vi "UHR-Fleezers Control (host) - 12.7.vi"() -> ()   [LabVIEW 2012] (continued)
        n1557 = Multiply(x=w2182, y="Number of F/B Scans (AOD)") -> (x*y=w2179:dbl)
        n1558 = Divide(x=w2179, y=60.0) -> (x/y=→"Time to Finish All (min)":dbl)
        n1559 = Add(x="Trap 2 Bead Size (nm)", y="Trap 1 Bead Size (nm)") -> (x+y=w2223:dbl)
        n1560 = Divide(x=w2223, y=2.0) -> (x/y=w2217:dbl)
        n1561 = local read "Initial delta (MHz)"() -> (w2220:dbl)
        n1562 = Subtract(x=w2234, y=w2233) -> (x-y=w2231:dbl)
        n1563 = Subtract(x=w2235, y=w2236) -> (x-y=w2232:dbl)
        n1564 = Square(x=w2231) -> (x^2=w2230:dbl)
        n1565 = Square(x=w2232) -> (x^2=w2229:dbl)
        n1566 = Add(x=w2229, y=w2230) -> (x+y=w2228:dbl)
        n1567 = Square Root(x=w2228) -> (sqrt(x)=w2227:dbl)
        "Final delta (MHz)" <- w2227
        n1568 = Multiply(x=w2219, y=w2227) -> (x*y=w2226:dbl)
        n1569 = Multiply(x=w2220, y=w2219) -> (x*y=w2218:dbl)
        n1570 = Subtract(x=w2218, y=w2217) -> (x-y=→"Initial sep (nm)":dbl)
        n1571 = Subtract(x=w2226, y=w2217) -> (x-y=→"Final sep (nm)":dbl)
      }
      event "Freq or Amp switch first", "Swap F1 and F2", "Freq switch delay", "Amp switch delay": Value Change {
        n1572 = event-data() -> ()  [unwired: 7 out]
        n1573 = local read "Amp switch delay"() -> (w2252:u16)
        n1574 = local read "Swap F1 and F2"() -> (w2253:bool)
        n1575 = xnode "Read/Write Control"("FPGA VI Reference In"=w2256, "error in"=w2255, "Swap F1 and F2"=w2253, "Amp switch delay"=w2252) -> ("error out"=w2254:errorcluster)  [unwired: 1 out]
      }
      event "Scan steps (MCL)", "Number of scans (MCL)", "Scan Range (V)\n(of steps)", "2D or 1D Scan", "N APD Samp/step", "Fast Scan Dir", "Continuous MCL Scanning", "Scan lines (y)": Value Change {
        w2258 = 32767.0 ("y")
        n1576 = event-data() -> ()  [unwired: 7 out]
        n1577 = Select(t="Scan lines (y)", s="2D or 1D Scan", f="Number of scans (MCL)") -> (s? t:f=w2263:u64)
        n1578 = Decrement(x="Scan steps (MCL)") -> (x-1=w2279:u64)
        n1579 = Divide(x="Scan Range (V)\n(of steps)", y=w2279) -> (x/y=w2278:dbl)
        "Desired Scan Incr (V)" <- w2278
        n1580 = local read "APD Integration Time (s)"() -> (w2271:dbl)
        n1581 = Multiply(x=w2278, y=w2258) -> (x*y=w2287:dbl)
        n1582 = Divide(x=w2287, y=10.0) -> (x/y=w2277:dbl)
        "Desired incr (int)" <- w2277
        n1583 = local read "Update Count (MCL)"() -> (w2283:u32)
        n1584 = Round Toward -Infinity(1:w2277) -> (0:w2286:dbl)
        n1585 = To Word Integer(number=w2286) -> (16bit integer=w2261:i16)
        "Actual Incr. int (MCL)" <- w2261
        n1586 = Multiply(x=w2271, y=40000000.0) -> (x*y=w2284:dbl)
        n1587 = Divide(x=w2284, y=w2283) -> (x/y=w2282:dbl)
        n1588 = Multiply(x=i16 10, y=w2261) -> (x*y=w2259:i16)
        n1589 = Multiply(x="N APD Samp/step", y=w2282) -> (x*y=w2281:dbl)
        "Cycles/step (MCL)" <- w2281
        n1590 = Divide(x=w2259, y=w2258) -> (x/y=→"Actual MCL Inc (V)":dbl)
        n1591 = Multiply(x="N APD Samp/step", y="Scan steps (MCL)") -> (x*y=w2273:dbl)
        n1592 = local read "APD Samples/FIFO Acq."() -> (w2270:dbl)
        n1593 = Multiply(x=w2273, y=u64 2) -> (x*y=w2272:dbl)
        "Data points/scan (f+b)" <- w2272
        n1594 = Multiply(x=w2272, y=w2263) -> (x*y=w2290:dbl)
        "Data points/scans (MCL)" <- w2290
        n1595 = Multiply(x=w2271, y=w2272) -> (x*y=w2264:dbl)
        "Time/f+b scan (s) (MCL)" <- w2264
        n1596 = Divide(x=w2290, y=w2270) -> (x/y=→"N sets should be saved (MCL)":dbl)
        n1597 = Multiply(x=w2264, y=w2263) -> (x*y=→"Total Time (s)":dbl)
        n1598 = Not(x="Fast Scan Dir") -> (.not. x?=w2268:bool)
        n1599 = xnode "Read/Write Control"("FPGA VI Reference In"=w2294, "error in"=w2293, "Scan steps (MCL)"="Scan steps (MCL)", "Number of scans (MCL)"=w2263, "Cycles per step (MCL)"=w2281, "Scan freq.  increment (MCL)"=w2261, "1D or 2D Scan?"="2D or 1D Scan", "MCL Scan Axis"=w2268, "Cont. Scan (MCL)"="Continuous MCL Scanning") -> ("error out"=w2292:errorcluster)  [unwired: 1 out]
      }
      event "Read Cal": Value Change {
        w2296 = 1000.0 ("y")
        n1600 = event-data() -> ()  [unwired: 7 out]
        n1601 = local read "Save file name"() -> (w2321:path)
        n1602 = local write "Read Cal"(FALSE ("Read Cal")) -> ()
        n1603 = Strip Path(path=w2321) -> (stripped path=w2320:path)  [unwired: 1 out]
        n1604 = Path To String(path=w2320) -> (string=w2319:string)
        n1605 = Concatenate Strings(w2319, "\\current.cal" ("string")) -> (w2317:string)
        n1606 = String To Path(string=w2317) -> (path=w2316:path)
        n1607 = Open/Create/Replace File(file path (use dialog)=w2316, operation (0:open)=T29."open", access (0:read/write)=enum16{"read/write", "read-only", "write-only"}."read-only") -> (refnum out=w2324:refnum<file>, error out=w2310:errorcluster)  [unwired: 1 in, 3 out]
        n1608 = Deny Access(4:w2310, 7:w2324) -> (0:w2309:errorcluster, 3:w2315:refnum<file>)  [unwired: 1 out]
        n1609 = Read from Binary File(5:0.0, 8:w2309, 9:T28."big-endian, network order" ("byte order (0:big-endian, network order)"), 10:-1 ("count (1)"), 11:w2315) -> (0:w2308:errorcluster, 2:w2306:dbl[], 3:w2311:refnum<file>)  [unwired: 2 out]
        n1610 = Array To Cluster(array=w2306) -> (cluster=w2305:T31)
        n1611 = Unbundle(w2305) -> ("[0]"=w2304:dbl, "[1]"=w2303:dbl, "[2]"=w2302:dbl, "[3]"=w2301:dbl, "[4]"=w2300:dbl, "[5]"=w2299:dbl)
        n1612 = Close File(refnum=w2311, error in=w2308) -> (error out=→"Read cal error":errorcluster)  [unwired: 1 out]
        n1613 = Multiply(x=w2299, y=w2296) -> (x*y=w2297:dbl)
        n1614 = local write "T2 kappa_x (pN/nm)"(w2301) -> ()
        n1615 = local write "T1 kappa_x (pN/nm)"(w2302) -> ()
        n1616 = local write "T1 alpha_x (nm/V)"(w2304) -> ()
        n1617 = local write "T2 alpha_x (nm/V)"(w2303) -> ()
        n1618 = Multiply(x=w2300, y=w2296) -> (x*y=w2298:dbl)
        n1619 = local write "T1 offset_x (mV)"(w2298) -> ()
        n1620 = local write "T2 offset_x (mV)"(w2297) -> ()
      }
      event "Abort MCL Scan": Value Change {
        n1621 = event-data() -> ()  [unwired: 7 out]
        n1622 = local write "MCL Scanning"(FALSE ("MCL Scanning")) -> ()
        n1623 = xnode "Read/Write Control"("FPGA VI Reference In"=w2329, "error in"=w2328, "Abort scan (MCL)"="Abort MCL Scan") -> ("error out"=w2327:errorcluster)  [unwired: 1 out]
      }
      event "Update Count (MCL)": Value Change {
        n1624 = event-data() -> ()  [unwired: 7 out]
        n1625 = xnode "Read/Write Control"("FPGA VI Reference In"=w2333, "error in"=w2332, "MCL count"="Update Count (MCL)") -> ("error out"=w2331:errorcluster)  [unwired: 1 out]
      }
      event "+ phase (MCL)", "- phase (MCL)": Value Change {
        n1626 = event-data() -> ()  [unwired: 7 out]
        n1627 = Or(x="- phase (MCL)", y="+ phase (MCL)") -> (x .or. y?=w2336:bool)
        n1628 = Negate(x="Phase adjust (MCL)") -> (-x=w2342:i16)
        n1629 = Select(t=w2342, s="+ phase (MCL)", f="Phase adjust (MCL)") -> (s? t:f=w2340:i16)
        n1630 = xnode "Read/Write Control"("FPGA VI Reference In"=w2344, "error in"=w2343, "Phase count adjustment (MCL)"=w2340) -> ("FPGA VI Reference Out"=w2337:T20, "error out"=w2338:errorcluster)
        n1631 = xnode "Read/Write Control"("FPGA VI Reference In"=w2337, "error in"=w2338, "+ phase (MCL)"=w2336) -> ("error out"=w2335:errorcluster)  [unwired: 1 out]
      }
      event "Abort AOD Scan": Value Change {
        n1632 = event-data() -> ()  [unwired: 7 out]
        n1633 = xnode "Read/Write Control"("FPGA VI Reference In"=w2348, "error in"=w2347, "Abort scan"="Abort AOD Scan") -> ("error out"=w2346:errorcluster)  [unwired: 1 out]
      }
      event "Continuous AOD Scanning": Value Change {
        n1634 = event-data() -> ()  [unwired: 7 out]
        n1635 = xnode "Read/Write Control"("FPGA VI Reference In"=w2352, "error in"=w2351, "Cont. Scan"="Continuous AOD Scanning") -> ("error out"=w2350:errorcluster)  [unwired: 1 out]
      }
      event "Index": Value Change {
        n1636 = event-data() -> ()  [unwired: 7 out]
        n1637 = call "Create new save file.vi"("Insert"="", "Ext"=".dat" ("string"), "Index In"="Index") -> ("Path Out"=→"Save file name":path, "Index Out"=w2353:dbl)
        "Save index" <- w2353
        n1638 = local write "Index"(w2353) -> ()
      }
      event "AO1", "AO2": Value Change {
        w2368 = 10.0 ("y")
        w2367 = 32767.0 ("y")
        n1639 = event-data() -> ()  [unwired: 7 out]
        n1640 = local read "AO2"() -> (w2366:dbl)
        n1641 = local read "AO1"() -> (w2363:dbl)
        n1642 = Multiply(x=w2363, y=w2367) -> (x*y=w2362:dbl)
        n1643 = Multiply(x=w2366, y=w2367) -> (x*y=w2365:dbl)
        n1644 = Divide(x=w2362, y=w2368) -> (x/y=w2361:dbl)
        n1645 = Divide(x=w2365, y=w2368) -> (x/y=w2364:dbl)
        n1646 = To Word Integer(number=w2361) -> (16bit integer=w2369:i16)
        n1647 = To Word Integer(number=w2364) -> (16bit integer=w2370:i16)
        n1648 = xnode "Read/Write Control"("FPGA VI Reference In"=w2360, "error in"=w2359, "AO1"=w2369, "AO2"=w2370) -> ("error out"=w2358:errorcluster)  [unwired: 1 out]
      }
      event "Inject Pump 1": Value Change {
        n1649 = event-data() -> ()  [unwired: 7 out]
        n1650 = local read "Use Harvard pumps\nfor beads (else Chemyx)"() -> (w2372:bool)
        n1651 = case shown="True" w2372 {
          tunnel: "Inject Pump 1" -> [w2376 w2414]
          tunnel: w2371 -> [_ w2415]
          frame False {
            n1652 = local read "Pump write delay (ms)"() -> (w2375:dbl)
            n1653 = local read "Chemyx Syringe Pump Serial Port"() -> (w2374:refnum<visa-resource-name>)
            n1654 = case shown="True" w2376 {
              tunnel: w2375 -> [w2382 w2396]
              tunnel: w2374 -> [w2379 w2395]
              frame False {
                n1655 = flat-sequence {
                  tunnel: w2379 -> [w2383]
                  tunnel: [w2383] -> w2380
                  tunnel: w2382 -> [_]
                  tunnel: [w2386] -> w2381
                  tunnel: w2380 -> [w2386]
                  tunnel: w2381 -> [w2387]
                  tunnel: [w2387] -> w2377
                  tunnel: [w2389] -> w2378
                  tunnel: w2377 -> [w2389]
                  tunnel: w2378 -> [w2391]
                  frame #0 {
                    n1656 = call "Write to pump.vi"("string"="enter pump1", "VISA resource name"=w2383) -> ()  [unwired: 1 out]
                  }
                  frame #1 {
                    n1657 = Wait (ms)(milliseconds to wait="Pump pause delay (ms)") -> ()  [unwired: 1 out]
                  }
                  frame #2 {
                    n1658 = call "Write to pump.vi"("string"="stop", "VISA resource name"=w2387) -> ()  [unwired: 1 out]
                  }
                  frame #3 {
                    n1659 = Wait (ms)(milliseconds to wait=u32 500) -> ()  [unwired: 1 out]
                  }
                  frame #4 {
                    n1660 = call "Write to pump.vi"("string"="stop", "VISA resource name"=w2391) -> ()  [unwired: 1 out]
                  }
                }
              }
              frame True {
                n1661 = flat-sequence {
                  tunnel: w2395 -> [w2405]
                  tunnel: w2396 -> [w2400]
                  tunnel: w2396 -> [w2407]
                  tunnel: w2395 -> [w2408]
                  tunnel: [w2408] -> w2393
                  tunnel: [w2410] -> w2394
                  tunnel: w2393 -> [w2410]
                  tunnel: w2394 -> [w2412]
                  frame #0 {
                    n1662 = local read "All Pump Parameters"() -> (w2399:T5)
                    n1663 = Unbundle By Name(w2399) -> ("Pump 1"=w2406:T32)
                    n1664 = call "Set pump parameters.vi"("Pump write delay (ms)"=w2400, "Volume (uL)"="Ch 1 Inject Volume (uL)", "Rate (uL/h)"="Ch 1 Inject Rate (ul/h)", "Units"=4.0, "Pump #"=1.0, "Pump Parameters In"=w2406, "VISA resource name"=w2405) -> ("Pump Parameters Out"=w2398:T32)  [unwired: 3 in]
                    n1665 = Bundle By Name(cluster=w2399, "Pump 1"=w2398) -> (w2397:T5)
                    n1666 = local write "All Pump Parameters"(w2397) -> ()
                  }
                  frame #1 {
                    n1667 = Wait (ms)(milliseconds to wait=w2407) -> ()  [unwired: 1 out]
                  }
                  frame #2 {
                    n1668 = call "Write to pump.vi"("string"="start", "VISA resource name"=w2408) -> ()  [unwired: 1 out]
                  }
                  frame #3 {
                    n1669 = Wait (ms)(milliseconds to wait=u32 500) -> ()  [unwired: 1 out]
                  }
                  frame #4 {
                    n1670 = call "Write to pump.vi"("string"="start", "VISA resource name"=w2412) -> ()  [unwired: 1 out]
                  }
                }
              }
            }
          }
          frame True {
            n1671 = case shown="False" w2414 {
              tunnel: w2415 -> [w2416 w2426]
              frame False {
                n1672 = flat-sequence {
                  tunnel: w2416 -> [w2418]
                  frame #0 {
                    n1673 = local write "Flushing P1"(FALSE ("Flushing P1")) -> ()
                    n1674 = Concatenate Strings("stop" ("string"), "\r") -> (w2420:string)
                    n1675 = VISA Write(VISA resource name=w2418, write buffer=w2420) -> ()  [unwired: 1 in, 3 out]
                  }
                  frame #1 {
                    n1676 = property on="Clear Volume P1" class="Bool (strict)"("Val(Sgnl)"=TRUE ("Value (Signaling)")) -> ()  [unwired: 2 in, 2 out]
                  }
                }
              }
              frame True {
                n1677 = local read "Normal Flow Rate (ul/h) P1"() -> (w2424:dbl)
                n1678 = Number To Decimal String(number=w2424) -> (decimal integer string=w2430:string)  [unwired: 1 in]
                n1679 = Concatenate Strings("irate  " ("string"), w2430, " u/h" ("string"), "\r") -> (w2428:string)
                n1680 = VISA Write(VISA resource name=w2426, write buffer=w2428) -> (VISA resource name out=w2425:refnum<visa-resource-name>)  [unwired: 1 in, 2 out]
                n1681 = Concatenate Strings("irun" ("string"), "\r") -> (w2432:string)
                n1682 = VISA Write(VISA resource name=w2425, write buffer=w2432) -> ()  [unwired: 1 in, 3 out]
              }
            }
          }
        }
      }
      event "Inject Pump 3": Value Change {
        n1683 = event-data() -> ()  [unwired: 7 out]
        n1684 = local read "Use Harvard pumps\nfor beads (else Chemyx)"() -> (w2435:bool)
        n1685 = case shown="True" w2435 {
          tunnel: "Inject Pump 3" -> [w2439 w2478]
          tunnel: w2434 -> [_ w2477]
          frame False {
            n1686 = local read "Pump write delay (ms)"() -> (w2438:dbl)
            n1687 = case shown="True" w2439 {
              tunnel: w2438 -> [w2445 w2459]
              tunnel: "Chemyx Syringe Pump Serial Port" -> [w2442 w2458]
              frame False {
                n1688 = flat-sequence {
                  tunnel: w2442 -> [w2446]
                  tunnel: [w2446] -> w2443
                  tunnel: w2445 -> [_]
                  tunnel: [w2449] -> w2444
                  tunnel: w2443 -> [w2449]
                  tunnel: w2444 -> [w2450]
                  tunnel: [w2450] -> w2440
                  tunnel: [w2452] -> w2441
                  tunnel: w2440 -> [w2452]
                  tunnel: w2441 -> [w2454]
                  frame #0 {
                    n1689 = call "Write to pump.vi"("string"="enter pump3", "VISA resource name"=w2446) -> ()  [unwired: 1 out]
                  }
                  frame #1 {
                    n1690 = local read "Pump pause delay (ms)"() -> (w2448:u32)
                    n1691 = Wait (ms)(milliseconds to wait=w2448) -> ()  [unwired: 1 out]
                  }
                  frame #2 {
                    n1692 = call "Write to pump.vi"("string"="stop", "VISA resource name"=w2450) -> ()  [unwired: 1 out]
                  }
                  frame #3 {
                    n1693 = Wait (ms)(milliseconds to wait=u32 0) -> ()  [unwired: 1 out]
                  }
                  frame #4 {
                    n1694 = call "Write to pump.vi"("string"="stop", "VISA resource name"=w2454) -> ()  [unwired: 1 out]
                  }
                }
              }
              frame True {
                n1695 = flat-sequence {
                  tunnel: w2458 -> [w2468]
                  tunnel: w2459 -> [w2463]
                  tunnel: w2459 -> [w2470]
                  tunnel: w2458 -> [w2471]
                  tunnel: [w2471] -> w2457
                  tunnel: [w2474] -> w2456
                  tunnel: w2457 -> [w2474]
                  tunnel: w2456 -> [w2475]
                  frame #0 {
                    n1696 = local read "All Pump Parameters"() -> (w2462:T5)
                    n1697 = Unbundle By Name(w2462) -> ("Pump 3"=w2469:T32)
                    n1698 = call "Set pump parameters.vi"("Pump write delay (ms)"=w2463, "Volume (uL)"="Ch 3 Inject Volume (uL)", "Rate (uL/h)"="Ch 3 Inject Rate (ul/h)", "Units"=4.0, "Pump #"=3.0, "Pump Parameters In"=w2469, "VISA resource name"=w2468) -> ("Pump Parameters Out"=w2461:T32)  [unwired: 3 in]
                    n1699 = Bundle By Name(cluster=w2462, "Pump 3"=w2461) -> (w2460:T5)
                    n1700 = local write "All Pump Parameters"(w2460) -> ()
                  }
                  frame #1 {
                    n1701 = Wait (ms)(milliseconds to wait=w2470) -> ()  [unwired: 1 out]
                  }
                  frame #2 {
                    n1702 = call "Write to pump.vi"("string"="start", "VISA resource name"=w2471) -> ()  [unwired: 1 out]
                  }
                  frame #3 {
                    n1703 = Wait (ms)(milliseconds to wait=u32 500) -> ()  [unwired: 1 out]
                  }
                  frame #4 {
                    n1704 = call "Write to pump.vi"("string"="start", "VISA resource name"=w2475) -> ()  [unwired: 1 out]
                  }
                }
              }
            }
          }
          frame True {
            n1705 = case shown="False" w2478 {
              tunnel: w2477 -> [w2479 w2486]
              frame False {
                n1706 = flat-sequence {
                  tunnel: w2479 -> [w2481]
                  frame #0 {
                    n1707 = local write "Flushing P3"(FALSE ("Flushing P3")) -> ()
                    n1708 = Concatenate Strings("stop" ("string"), "\r") -> (w2483:string)
                    n1709 = VISA Write(VISA resource name=w2481, write buffer=w2483) -> ()  [unwired: 1 in, 3 out]
                  }
                  frame #1 {
                    n1710 = property on="Clear Volume P3" class="Bool (strict)"("Val(Sgnl)"=TRUE ("Value (Signaling)")) -> ()  [unwired: 2 in, 2 out]
                  }
                }
              }
              frame True {
                n1711 = local read "Normal Flow Rate (ul/h) P3"() -> (w2487:dbl)
                n1712 = Number To Decimal String(number=w2487) -> (decimal integer string=w2493:string)  [unwired: 1 in]
                n1713 = Concatenate Strings("irate  " ("string"), w2493, " u/h" ("string"), "\r") -> (w2491:string)
                n1714 = VISA Write(VISA resource name=w2486, write buffer=w2491) -> (VISA resource name out=w2489:refnum<visa-resource-name>)  [unwired: 1 in, 2 out]
                n1715 = Concatenate Strings("irun" ("string"), "\r") -> (w2495:string)
                n1716 = VISA Write(VISA resource name=w2489, write buffer=w2495) -> ()  [unwired: 1 in, 3 out]
              }
            }
          }
        }
      }
      event "Inject Pump 2": Value Change {
        n1717 = event-data() -> ()  [unwired: 7 out]
        n1718 = local read "Pump write delay (ms)"() -> (w2499:dbl)
        n1719 = flat-sequence {
          tunnel: w2497 -> [w2512]
          tunnel: w2499 -> [w2508]
          tunnel: "Inject Pump 2" -> [_]
          tunnel: w2499 -> [w2514]
          tunnel: w2497 -> [w2515]
          frame #0 {
            n1720 = local read "All Pump Parameters"() -> (w2507:T5)
            n1721 = Multiply(x=60.0, y="Flush Center Ch Rate (ul/m)") -> (x*y=w2504:dbl)
            n1722 = Unbundle By Name(w2507) -> ("Pump 2"=w2513:T32)
            n1723 = call "Set pump parameters.vi"("Pump write delay (ms)"=w2508, "Volume (uL)"="Flush Center Ch Volume (uL)", "Rate (uL/h)"=w2504, "Units"=3.0, "Pump #"=2.0, "Pump Parameters In"=w2513, "VISA resource name"=w2512) -> ("Pump Parameters Out"=w2506:T32)  [unwired: 3 in]
            n1724 = Bundle By Name(cluster=w2507, "Pump 2"=w2506) -> (w2505:T5)
            n1725 = local write "All Pump Parameters"(w2505) -> ()
            n1726 = Add(x="Flush Center Ch Volume (uL)", y="Total Volume\nFlushed (uL)") -> (x+y=w2501:dbl)
            n1727 = local write "Total Volume\nFlushed (uL)"(w2501) -> ()
          }
          frame #1 {
            n1728 = Wait (ms)(milliseconds to wait=w2514) -> ()  [unwired: 1 out]
          }
          frame #2 {
            n1729 = call "Write to pump.vi"("string"="start", "VISA resource name"=w2515) -> ()  [unwired: 1 out]
          }
        }
        n1730 = local read "Chemyx Syringe Pump Serial Port"() -> (w2497:refnum<visa-resource-name>)
      }
      event "Sample Channel\nFlow": Value Change {
        n1731 = event-data() -> ()  [unwired: 7 out]
        n1732 = Select(t="irun" ("string"), s="Sample Channel\nFlow", f="stop" ("string")) -> (s? t:f=w2519:string)
        n1733 = Concatenate Strings(w2519, "\r") -> (w2522:string)
        n1734 = VISA Write(VISA resource name=w2517, write buffer=w2522) -> ()  [unwired: 1 in, 3 out]
      }
      event "Start Flow": Value Change {
        n1735 = event-data() -> ()  [unwired: 7 out]
        n1736 = local write "Sample Channel\nFlow"(TRUE ("Sample Channel\nFlow")) -> ()
        n1737 = local write "Start Flow"(FALSE ("Start Flow")) -> ()
        n1738 = Concatenate Strings("irun" ("string"), "\r") -> (w2528:string)
        n1739 = VISA Write(VISA resource name=w2524, write buffer=w2528) -> ()  [unwired: 1 in, 3 out]
      }
      event "Stop Flow": Value Change {
        w2530 = FALSE ("Stop Flow")
        n1740 = event-data() -> ()  [unwired: 7 out]
        n1741 = local write "Stop Flow"(w2530) -> ()
        n1742 = local write "Sample Channel\nFlow"(w2530) -> ()
        n1743 = Concatenate Strings("stop" ("string"), "\r") -> (w2533:string)
        n1744 = VISA Write(VISA resource name=w2531, write buffer=w2533) -> ()  [unwired: 1 in, 3 out]
      }
      event "Flow rate (uL/h)": Value Change {
        n1745 = event-data() -> ()  [unwired: 7 out]
        n1746 = Number To Decimal String(number="Flow rate (uL/h)") -> (decimal integer string=w2540:string)  [unwired: 1 in]
        n1747 = Concatenate Strings("irate  " ("string"), w2540, " u/h" ("string"), "\r") -> (w2539:string)
        n1748 = VISA Write(VISA resource name=w2536, write buffer=w2539) -> ()  [unwired: 1 in, 3 out]
      }
      event "Flush Sample": Value Change {
        n1749 = event-data() -> ()  [unwired: 7 out]
        n1750 = flat-sequence {
          tunnel: w2545 -> [w2573]
          tunnel: [w2553] -> w2544
          tunnel: [w2547] -> w2542
          tunnel: w2544 -> [w2577]
          tunnel: [w2577] -> w2543
          tunnel: w2542 -> [w2576]
          tunnel: w2543 -> [w2582]
          frame #0 {
            # "set paramaters (rate, volume) for flush, clear volume"
            n1751 = Number To Decimal String(number="Flush rate (uL/m)") -> (decimal integer string=w2569:string)  [unwired: 1 in]
            n1752 = Concatenate Strings("irate  " ("string"), w2569, " u/m" ("string"), "\r") -> (w2571:string)
            n1753 = VISA Write(VISA resource name=w2573, write buffer=w2571) -> (VISA resource name out=w2567:refnum<visa-resource-name>)  [unwired: 1 in, 2 out]
            n1754 = Reciprocal(x="Flush rate (uL/m)") -> (1/x=w2550:dbl)
            n1755 = Number To Decimal String(number="Volume (uL)") -> (decimal integer string=w2558:string)  [unwired: 1 in]
            n1756 = Multiply(x="Volume (uL)", y=w2550) -> (x*y=w2549:dbl)
            n1757 = Concatenate Strings("tvolume  " ("string"), w2558, " u" ("string"), "\r") -> (w2556:string)
            n1758 = Multiply(x=w2549, y=60000.0) -> (x*y=w2547:dbl)
            n1759 = VISA Write(VISA resource name=w2567, write buffer=w2556) -> (VISA resource name out=w2555:refnum<visa-resource-name>)  [unwired: 1 in, 2 out]
            n1760 = Concatenate Strings("cvolume" ("string"), "\r") -> (w2554:string)
            n1761 = VISA Write(VISA resource name=w2555, write buffer=w2554) -> (VISA resource name out=w2565:refnum<visa-resource-name>)  [unwired: 1 in, 2 out]
            n1762 = Concatenate Strings("irun" ("string"), "\r") -> (w2563:string)
            n1763 = VISA Write(VISA resource name=w2565, write buffer=w2563) -> (VISA resource name out=w2553:refnum<visa-resource-name>)  [unwired: 1 in, 2 out]
          }
          frame #1 {
            # "Have to wait until\nflow is done to reset\nrate"
            n1764 = Add(x=w2576, y=100.0) -> (x+y=w2575:dbl)
            n1765 = Wait (ms)(milliseconds to wait=w2575) -> ()  [unwired: 1 out]
          }
          frame #2 {
            # "reset flow rate to usual flow rate"
            n1766 = local read "Flow rate (uL/h)"() -> (w2588:dbl)
            n1767 = Number To Decimal String(number=w2588) -> (decimal integer string=w2586:string)  [unwired: 1 in]
            n1768 = Concatenate Strings("irate  " ("string"), w2586, " u/h" ("string"), "\r") -> (w2584:string)
            n1769 = VISA Write(VISA resource name=w2582, write buffer=w2584) -> (VISA resource name out=w2578:refnum<visa-resource-name>)  [unwired: 1 in, 2 out]
            n1770 = Concatenate Strings("cvolume" ("string"), "\r") -> (w2579:string)
            n1771 = VISA Write(VISA resource name=w2578, write buffer=w2579) -> ()  [unwired: 1 in, 3 out]
          }
        }
      }
      event "Flush Pump 3": Value Change {
        n1772 = event-data() -> ()  [unwired: 7 out]
        n1773 = flat-sequence {
          tunnel: w2589 -> [w2592]
          frame #0 {
            # "set paramaters (rate, volume) for flush, clear volume"
            n1774 = Number To Decimal String(number="Flush rate (uL/m) P3") -> (decimal integer string=w2614:string)  [unwired: 1 in]
            n1775 = local write "Inject Pump 3"(TRUE ("Inject Pump 3")) -> ()
            n1776 = Concatenate Strings("irate  " ("string"), w2614, " u/m" ("string"), "\r") -> (w2616:string)
            n1777 = VISA Write(VISA resource name=w2592, write buffer=w2616) -> (VISA resource name out=w2612:refnum<visa-resource-name>)  [unwired: 1 in, 2 out]
            n1778 = Reciprocal(x="Flush rate (uL/m) P3") -> (1/x=w2596:dbl)
            n1779 = Number To Decimal String(number="Volume (uL) P3") -> (decimal integer string=w2603:string)  [unwired: 1 in]
            n1780 = Multiply(x="Volume (uL) P3", y=w2596) -> (x*y=w2595:dbl)
            n1781 = Concatenate Strings("tvolume  " ("string"), w2603, " u" ("string"), "\r") -> (w2601:string)
            n1782 = Multiply(x=w2595, y=60.0) -> (x*y=→"HP3 Flush Time (s)":dbl)
            n1783 = VISA Write(VISA resource name=w2612, write buffer=w2601) -> (VISA resource name out=w2600:refnum<visa-resource-name>)  [unwired: 1 in, 2 out]
            n1784 = Concatenate Strings("cvolume" ("string"), "\r") -> (w2599:string)
            n1785 = VISA Write(VISA resource name=w2600, write buffer=w2599) -> (VISA resource name out=w2610:refnum<visa-resource-name>)  [unwired: 1 in, 2 out]
            n1786 = Concatenate Strings("irun" ("string"), "\r") -> (w2608:string)
            n1787 = VISA Write(VISA resource name=w2610, write buffer=w2608) -> ()  [unwired: 1 in, 3 out]
          }
          frame #1 {
            "Flushing P3" <- TRUE ("Flushing P3")
          }
        }
      }
      event "Flush Pump 1": Value Change {
        n1788 = event-data() -> ()  [unwired: 7 out]
        n1789 = flat-sequence {
          tunnel: [w2630] -> w2620
          tunnel: w2619 -> [w2623]
          tunnel: w2620 -> [_]
          frame #0 {
            # "set paramaters (rate, volume) for flush, clear volume"
            n1790 = local write "Inject Pump 1"(TRUE ("Inject Pump 1")) -> ()
            n1791 = Number To Decimal String(number="Flush rate (uL/m) P1") -> (decimal integer string=w2646:string)  [unwired: 1 in]
            n1792 = Concatenate Strings("irate  " ("string"), w2646, " u/m" ("string"), "\r") -> (w2648:string)
            n1793 = VISA Write(VISA resource name=w2623, write buffer=w2648) -> (VISA resource name out=w2644:refnum<visa-resource-name>)  [unwired: 1 in, 2 out]
            n1794 = Reciprocal(x="Flush rate (uL/m) P1") -> (1/x=w2627:dbl)
            n1795 = Number To Decimal String(number="Volume (uL) P1") -> (decimal integer string=w2635:string)  [unwired: 1 in]
            n1796 = Multiply(x="Volume (uL) P1", y=w2627) -> (x*y=w2626:dbl)
            n1797 = Concatenate Strings("tvolume  " ("string"), w2635, " u" ("string"), "\r") -> (w2633:string)
            n1798 = Multiply(x=w2626, y=60.0) -> (x*y=→"HP1 Flush Time (s)":dbl)
            n1799 = VISA Write(VISA resource name=w2644, write buffer=w2633) -> (VISA resource name out=w2632:refnum<visa-resource-name>)  [unwired: 1 in, 2 out]
            n1800 = Concatenate Strings("cvolume" ("string"), "\r") -> (w2631:string)
            n1801 = VISA Write(VISA resource name=w2632, write buffer=w2631) -> (VISA resource name out=w2642:refnum<visa-resource-name>)  [unwired: 1 in, 2 out]
            n1802 = Concatenate Strings("irun" ("string"), "\r") -> (w2640:string)
            n1803 = VISA Write(VISA resource name=w2642, write buffer=w2640) -> (VISA resource name out=w2630:refnum<visa-resource-name>)  [unwired: 1 in, 2 out]
          }
          frame #1 {
            "Flushing P1" <- TRUE ("Flushing P3")
          }
        }
      }
      event "Clear Volume": Value Change {
        n1804 = event-data() -> ()  [unwired: 7 out]
        n1805 = Concatenate Strings("cvolume" ("string"), "\r") -> (w2652:string)
        n1806 = VISA Write(VISA resource name=w2651, write buffer=w2652) -> ()  [unwired: 1 in, 3 out]
      }
      event "Clear Volume P3": Value Change {
        n1807 = event-data() -> ()  [unwired: 7 out]
        n1808 = Concatenate Strings("cvolume" ("string"), "\r") -> (w2658:string)
        n1809 = VISA Write(VISA resource name=w2657, write buffer=w2658) -> ()  [unwired: 1 in, 3 out]
        n1810 = local write "Clear Volume P3"(FALSE ("Clear Volume P3")) -> ()
      }
      event "Clear Volume P1": Value Change {
        n1811 = event-data() -> ()  [unwired: 7 out]
        n1812 = Concatenate Strings("cvolume" ("string"), "\r") -> (w2663:string)
        n1813 = local write "Clear Volume P1"(FALSE ("Clear Volume P1")) -> ()
        n1814 = VISA Write(VISA resource name=w2662, write buffer=w2663) -> ()  [unwired: 1 in, 3 out]
      }
      event "Display On P3": Value Change {
        n1815 = event-data() -> ()  [unwired: 7 out]
        n1816 = Select(t="dim 100", s="Display On P3", f="dim 0") -> (s? t:f=w2669:string)
        n1817 = Concatenate Strings(w2669, "\r") -> (w2671:string)
        n1818 = VISA Write(VISA resource name=w2666, write buffer=w2671) -> ()  [unwired: 1 in, 3 out]
      }
      event "Display On P1": Value Change {
        n1819 = event-data() -> ()  [unwired: 7 out]
        n1820 = Select(t="dim 100", s="Display On P1", f="dim 0") -> (s? t:f=w2676:string)
        n1821 = Concatenate Strings(w2676, "\r") -> (w2678:string)
        n1822 = VISA Write(VISA resource name=w2673, write buffer=w2678) -> ()  [unwired: 1 in, 3 out]
      }
      event "Retract Pump 3": Value Change {
        n1823 = event-data() -> ()  [unwired: 7 out]
        n1824 = local write "Retract Pump 3"(FALSE ("Retract Pump 3")) -> ()
        n1825 = case shown="True" "Retract Pump 3" {
          tunnel: w2680 -> [_ w2683]
          frame False {
          }
          frame True {
            n1826 = Number To Decimal String(number="Retract Rate (uL/m)") -> (decimal integer string=w2701:string)  [unwired: 1 in]
            n1827 = Concatenate Strings("wrate  " ("string"), w2701, " u/m" ("string"), "\r") -> (w2703:string)
            n1828 = VISA Write(VISA resource name=w2683, write buffer=w2703) -> (VISA resource name out=w2694:refnum<visa-resource-name>)  [unwired: 1 in, 2 out]
            n1829 = Number To Decimal String(number="Retract Vol 3 (uL)") -> (decimal integer string=w2696:string)  [unwired: 1 in]
            n1830 = Concatenate Strings("tvolume  " ("string"), w2696, " u" ("string"), "\r") -> (w2693:string)
            n1831 = VISA Write(VISA resource name=w2694, write buffer=w2693) -> (VISA resource name out=w2689:refnum<visa-resource-name>)  [unwired: 1 in, 2 out]
            n1832 = Concatenate Strings("cvolume" ("string"), "\r") -> (w2690:string)
            n1833 = VISA Write(VISA resource name=w2689, write buffer=w2690) -> (VISA resource name out=w2684:refnum<visa-resource-name>)  [unwired: 1 in, 2 out]
            n1834 = Concatenate Strings("wrun" ("string"), "\r") -> (w2685:string)
            n1835 = VISA Write(VISA resource name=w2684, write buffer=w2685) -> ()  [unwired: 1 in, 3 out]
          }
        }
      }
      event "Retract Pump 1": Value Change {
        n1836 = event-data() -> ()  [unwired: 7 out]
        n1837 = local write "Retract Pump 1"(FALSE ("Retract Pump 1")) -> ()
        n1838 = case shown="True" "Retract Pump 1" {
          tunnel: w2705 -> [_ w2710]
          frame False {
          }
          frame True {
            n1839 = local read "Retract Rate (uL/m)"() -> (w2708:dbl)
            n1840 = Number To Decimal String(number=w2708) -> (decimal integer string=w2726:string)  [unwired: 1 in]
            n1841 = Concatenate Strings("wrate  " ("string"), w2726, " u/m" ("string"), "\r") -> (w2728:string)
            n1842 = VISA Write(VISA resource name=w2710, write buffer=w2728) -> (VISA resource name out=w2720:refnum<visa-resource-name>)  [unwired: 1 in, 2 out]
            n1843 = Number To Decimal String(number="Retract Vol 1 (uL)") -> (decimal integer string=w2722:string)  [unwired: 1 in]
            n1844 = Concatenate Strings("tvolume  " ("string"), w2722, " u" ("string"), "\r") -> (w2719:string)
            n1845 = VISA Write(VISA resource name=w2720, write buffer=w2719) -> (VISA resource name out=w2716:refnum<visa-resource-name>)  [unwired: 1 in, 2 out]
            n1846 = Concatenate Strings("cvolume" ("string"), "\r") -> (w2717:string)
            n1847 = VISA Write(VISA resource name=w2716, write buffer=w2717) -> (VISA resource name out=w2711:refnum<visa-resource-name>)  [unwired: 1 in, 2 out]
            n1848 = Concatenate Strings("wrun" ("string"), "\r") -> (w2712:string)
            n1849 = VISA Write(VISA resource name=w2711, write buffer=w2712) -> ()  [unwired: 1 in, 3 out]
          }
        }
      }
      event "Flip Green Filter": Value Change {
        n1850 = event-data() -> ()  [unwired: 7 out]
        n1851 = Not(x="Flip Green Filter") -> (.not. x?=w2730:bool)
        n1852 = local write "Flip Green Filter"(w2730) -> ()
        n1853 = flat-sequence {
          tunnel: w2738 -> [w2743]
          tunnel: w2737 -> [w2742]
          tunnel: [w2740] -> w2735
          tunnel: [w2739] -> w2734
          tunnel: [w2745] -> w2733
          tunnel: w2735 -> [w2745]
          tunnel: [w2744] -> w2732
          tunnel: w2734 -> [w2744]
          tunnel: w2733 -> [w2749]
          tunnel: w2732 -> [w2748]
          tunnel: [w2747] -> w2736
          frame #0 {
            n1854 = xnode "Read/Write Control"("FPGA VI Reference In"=w2743, "error in"=w2742, "Green Filter Flipper"=TRUE) -> ("FPGA VI Reference Out"=w2740:T20, "error out"=w2739:errorcluster)
          }
          frame #1 {
            n1855 = Wait (ms)(milliseconds to wait=u32 100) -> ()  [unwired: 1 out]
          }
          frame #2 {
            n1856 = xnode "Read/Write Control"("FPGA VI Reference In"=w2749, "error in"=w2748, "Green Filter Flipper"=FALSE) -> ("error out"=w2747:errorcluster)  [unwired: 1 out]
          }
        }
      }
      event "Pump 1 contents", "Pump 3 contents": Value Change {
        n1857 = event-data() -> ()  [unwired: 7 out]
        n1858 = local read "Pump 1 contents"() -> (→"Pump 1 cont disp":string)
        n1859 = local read "Pump 3 contents"() -> (→"Pump 3 cont disp":string)
      }
      event "Reset Trap Pos. FB": Value Change {
        n1860 = event-data() -> ()  [unwired: 7 out]
        n1861 = xnode "Read/Write Control"("FPGA VI Reference In"=w2755, "error in"=w2754, "Trap Pos. FB Reset"="Reset Trap Pos. FB") -> ()  [unwired: 2 out]
      }
      event "Rem fb disp offset": Value Change {
        n1862 = event-data() -> ()  [unwired: 7 out]
        n1863 = local write "Rem fb disp offset"(FALSE ("Rem fb disp offset")) -> ()
        n1864 = local read "Mean T1 Position (nm)"() -> (w2757:dbl)
        n1865 = local read "FB Trap Pos Offset"() -> (w2758:dbl)
        n1866 = Subtract(x=w2758, y=w2757) -> (x-y=w2756:dbl)
        n1867 = local write "FB Trap Pos Offset"(w2756) -> ()
      }
      event "Threshold (nm)": Value Change {
        n1868 = event-data() -> ()  [unwired: 7 out]
        n1869 = flat-sequence {
          tunnel: w2762 -> [w2770]
          tunnel: w2761 -> [w2769]
          tunnel: [w2763] -> w2760
          tunnel: w2760 -> [w2776]
          frame #0 {
            n1870 = xnode "Read/Write Control"("FPGA VI Reference In"=w2770, "error in"=w2769) -> ("FPGA VI Reference Out"=w2766:T20, "error out"=w2765:errorcluster, "FPGA TTrig Thresh"=w2767:i64)
            n1871 = local read "Threshold stored (nm)"() -> (w2775:dbl)
            n1872 = local read "Threshold (nm)"() -> (w2763:dbl)
            n1873 = local read "AOM X Cal (nm/MHz)"() -> (w2773:dbl)
            n1874 = Subtract(x=w2763, y=w2775) -> (x-y=w2774:dbl)
            n1875 = Divide(x=w2774, y=w2773) -> (x/y=w2771:dbl)
            n1876 = call "IR AOM freq to word.vi"("Frequency In (MHz)"=w2771) -> ("Frequency Word Out (double)"=w2772:dbl)
            n1877 = To Quad Integer(1:w2772) -> (0:w2768:i64)
            n1878 = Add(x=w2767, y=w2768) -> (x+y=w2764:i64)
            n1879 = xnode "Read/Write Control"("FPGA VI Reference In"=w2766, "error in"=w2765, "FPGA TTrig Thresh"=w2764) -> ()  [unwired: 2 out]
          }
          frame #1 {
            "Threshold stored (nm)" <- w2776
          }
        }
      }
      event "FB Trig Integrate": Value Change {
        n1880 = event-data() -> ()  [unwired: 7 out]
        n1881 = local read "FB Trig Integrate"() -> (w2778:u32)
        n1882 = xnode "Read/Write Control"("FPGA VI Reference In"=w2780, "error in"=w2779, "FB Trig Integrate"=w2778) -> ("error out"=w2777:errorcluster)  [unwired: 1 out]
      }
      event "11": Value Change {
        n1883 = event-data() -> ()  [unwired: 7 out]
        n1884 = local read "11"() -> (w2781:bool)
        n1885 = case shown="True" w2781 {
          frame False {
          }
          frame True {
            n1886 = local read "Messages"() -> (w2783:string)
            n1887 = call "Update messages.vi"("Message to add"="You kicked it up to 11!", "Old message string"=w2783) -> ("New message string"=w2784:string)
            n1888 = call <vilib>:"Beep.vi"() -> ()  [unwired: 12 in]
            n1889 = local write "Messages"(w2784) -> ()
          }
        }
      }
      event "Trap Pos. FB ON": Value Change {
        n1890 = event-data() -> ()  [unwired: 7 out]
        n1891 = xnode "Read/Write Control"("FPGA VI Reference In"=w2787, "error in"=w2786, "Force feedback"="Trap Pos. FB ON") -> ()  [unwired: 2 out]
      }
      event "Remove Action Offset": Value Change {
        n1892 = event-data() -> ()  [unwired: 7 out]
        n1893 = local write "Remove Action Offset"(FALSE ("Remove Action Offset")) -> ()
        n1894 = local read "Trap Pos. FB Mult Factor"() -> (w2792:i64)
        n1895 = local read "Trap Pos FB Action"() -> (w2790:i64)
        n1896 = local read "Trap Pos. FB Offset Factor"() -> (w2788:i64)
        n1897 = Multiply(x=w2792, y=w2790) -> (x*y=w2791:i64)
        n1898 = Add(x=w2791, y=w2788) -> (x+y=w2789:i64)
        n1899 = local write "Trap Pos. FB Offset Factor"(w2789) -> ()
        n1900 = xnode "Read/Write Control"("FPGA VI Reference In"=w2795, "error in"=w2794, "Trap Pos. FB Offset Factor"=w2789) -> ()  [unwired: 2 out]
      }
      event "Remove Unwinding Offset": Value Change {
        n1901 = event-data() -> ()  [unwired: 7 out]
        n1902 = local write "Remove Unwinding Offset"(FALSE ("Remove Action Offset")) -> ()
        n1903 = local read "Trap Pos. FB Mult Factor"() -> (w2807:i64)
        n1904 = local read "Trap Pos FB Action"() -> (w2805:i64)
        n1905 = local read "Trap Pos. FB Offset Factor"() -> (w2804:i64)
        n1906 = Multiply(x=w2807, y=w2805) -> (x*y=w2806:i64)
        n1907 = local read "Trap Pos. FB Mult Factor"() -> (w2803:i64)
        n1908 = Add(x=w2806, y=w2804) -> (x+y=w2797:i64)
        n1909 = Multiply(x=32768, y="factor") -> (x*y=w2800:dbl)
        n1910 = Multiply(x=w2800, y=w2803) -> (x*y=w2802:dbl)
        n1911 = Subtract(x=w2797, y=w2802) -> (x-y=w2801:dbl)
        n1912 = To Quad Integer(1:w2801) -> (0:w2796:i64)
        n1913 = xnode "Read/Write Control"("FPGA VI Reference In"=w2810, "error in"=w2809, "Trap Pos. FB Offset Factor"=w2796) -> ()  [unwired: 2 out]
        n1914 = local write "Trap Pos. FB Offset Factor"(w2796) -> ()
      }
      event "Trap Pos. FB Range", "Trap Pos. FB Gains", "Trap Pos. FB Mult Factor", "Trap Pos. FB Offset Factor", "Trap Pos FB Negate Action", "Trap Pos FB Monitor\nT1 or T2", "Differential FB?", "Negate Diff?": Value Change {
        n1915 = event-data() -> ()  [unwired: 7 out]
        n1916 = Unbundle By Name("Trap Pos. FB Gains") -> ("proportional gain (Kc)"=w2813:fxp<+/-,16,8>, "integral gain (Kc*Ts/Ti)"=w2812:fxp<+/-,16,8>, "derivative gain (Kc*Td/Ts)"=w2811:fxp<+/-,16,8>)
        n1917 = local read "Negate Diff?"() -> (w2818:bool)
        n1918 = Unbundle By Name("Trap Pos. FB Range") -> ("output high"=w2816:fxp<+/-,16,1>, "output low"=w2815:fxp<+/-,16,1>)
        n1919 = xnode "Read/Write Control"("FPGA VI Reference In"=w2826, "error in"=w2825, "FB2 output high"=w2816, "FB2 output low"=w2815, "P2"=w2813, "I2"=w2812, "D2"=w2811, "Trap Pos. FB Mult Factor"="Trap Pos. FB Mult Factor", "Trap Pos. FB Offset Factor"="Trap Pos. FB Offset Factor", "Trap Pos FB Negate Action"="Trap Pos FB Negate Action", "Trap Pos FB Monitor T1 or T2"="Trap Pos FB Monitor\nT1 or T2", "AI1 X Scale"="Trap Pos. AI1 X Pre-scale", "Negate Diff?"=w2818, "Diff FB Measurement?"="Differential FB?") -> ()  [unwired: 2 out]
      }
      event "Trap Pos FB SP", "Trap Pos FB SP 2", "Use SP 2": Value Change {
        n1920 = event-data() -> ()  [unwired: 7 out]
        n1921 = Select(t="Trap Pos FB SP 2", s="Use SP 2", f="Trap Pos FB SP") -> (s? t:f=w2827:fxp<+/-,16,1>)
        n1922 = xnode "Read/Write Control"("FPGA VI Reference In"=w2832, "error in"=w2831, "Trap Pos. FB SP"=w2827) -> ()  [unwired: 2 out]
      }
      event "Offset SP2 from SP1": Value Change {
        n1923 = event-data() -> ()  [unwired: 7 out]
        n1924 = local read "Trap Pos FB SP"() -> (w2835:fxp<+/-,16,1>)
        n1925 = Add(x=w2835, y="SP2 Offset") -> (x+y=w2833:fxp<+/-,16,1>)
        n1926 = property on="Trap Pos FB SP 2" class="DigNum (strict)"("Val(Sgnl)"=w2833) -> ()  [unwired: 2 in, 2 out]
        n1927 = local write "Offset SP2 from SP1"(FALSE ("Offset SP2 from SP1")) -> ()
      }
      event "Set Reading to\nSetpoint": Value Change {
        # "This is the actual PID input signal"
        n1928 = event-data() -> ()  [unwired: 7 out]
        n1929 = local write "Set Reading to\nSetpoint"(FALSE ("Set SP to Reading")) -> ()
        n1930 = xnode "Read/Write Control"("FPGA VI Reference In"=w2841, "error in"=w2840) -> ("FPGA VI Reference Out"=w2839:T20, "error out"=w2838:errorcluster, "Trap Pos FB Int-Norm Signal"=w2837:fxp<+/-,16,1>)
        n1931 = local read "Differential FB?"() -> (w2842:bool)
        n1932 = case shown="False" w2842 {
          tunnel: [w2847 w2854] -> w2844
          tunnel: w2837 -> [w2845 w2854]
          frame False {
            n1933 = local read "Trap Pos FB Monitor\nT1 or T2"() -> (w2850:bool)
            n1934 = local read "Trap X AI1 (DMA)"() -> (w2853:T13)
            n1935 = Unbundle By Name(w2853) -> ("Set 1"=w2852:fxp<+/-,16,1>, "Set 2"=w2851:fxp<+/-,16,1>)
            n1936 = Select(t=w2852, s=w2850, f=w2851) -> (s? t:f=w2849:fxp<+/-,16,1>)
            n1937 = Not(x="Set SP Using...") -> (.not. x?=w2846:bool)
            n1938 = Select(t=w2845, s=w2846, f=w2849) -> (s? t:f=w2847:fxp<+/-,16,1>)
          }
          frame True {
          }
        }
        n1939 = xnode "Read/Write Control"("FPGA VI Reference In"=w2839, "error in"=w2838, "Trap Pos. FB SP"=w2844) -> ()  [unwired: 2 out]
        n1940 = local write "Trap Pos FB SP"(w2844) -> ()
      }
      event "Trap Pos. FB Out Scale 2^n": Value Change {
        n1941 = event-data() -> ()  [unwired: 7 out]
        n1942 = Scale By Power Of 2(n="Trap Pos. FB Out Scale 2^n", x=ext 1.0) -> (x*2^n=w2855:ext)
        n1943 = property on="Trap Pos. FB Mult Factor" class="DigNum (strict)"("Val(Sgnl)"=w2855) -> ()  [unwired: 2 in, 2 out]
      }
      event "Trap Pos FB Int Count": Value Change {
        n1944 = event-data() -> ()  [unwired: 7 out]
        n1945 = xnode "Read/Write Control"("FPGA VI Reference In"=w2860, "error in"=w2859, "Trap Pos FB Int Count"="Trap Pos FB Int Count") -> ()  [unwired: 2 out]
      }
      event "Trap pos": Value Change {
        n1946 = event-data() -> ()  [unwired: 7 out]
        n1947 = case shown="True" "Trap pos" {
          frame False {
            n1948 = property on="Trap Delta Graph" class="WFGraph (strict)"("Visible"=TRUE) -> ()  [unwired: 2 in, 2 out]
            n1949 = property on="Saved trap pos" class="WFGraph (strict)"("Visible"=FALSE) -> ()  [unwired: 2 in, 2 out]
          }
          frame True {
            n1950 = property on="Saved trap pos" class="WFGraph (strict)"("Visible"=TRUE) -> ()  [unwired: 2 in, 2 out]
            n1951 = property on="Trap Delta Graph" class="WFGraph (strict)"("Visible"=FALSE) -> ()  [unwired: 2 in, 2 out]
          }
        }
      }
    }
    "error out 2" <- w1687
    n1952 = node-c288() -> ()  [unwired: 2 out]
  }
  n1953 = while "Duncan's play event loop" {
    stop <- w2867 stop-if-true
    n1954 = Create User Event(user event datatype=TRUE ("Boolean")) -> (user event=w2868:refnum<user-event>)  [unwired: 1 in, 1 out]
    n1955 = Create User Event(user event datatype=TRUE ("Boolean")) -> (user event=w2875:refnum<user-event>)  [unwired: 1 in, 1 out]
    n1956 = global write "Global for fluorescence simulation mean (30 samples), (power series).vi" "Red Signal"(w2868) -> ()
    n1957 = global write "Global for fluorescence simulation mean (30 samples), (power series).vi" "Green Signal"(w2875) -> ()
    n1958 = register-events(w2875, w2868) -> (reference out=w2874:refnum<event-registration>)  [unwired: 2 in, 1 out]
    n1959 = event shown="[1] \"Get Fluorophore\": Value Change" {
      selector: w2874 -> [_ _ _ _]
      dyn-events: _ -> [_ _ _ _]
      timeout: 100 -> [_ _ _ _]
      event Timeout {
        n1960 = event-data() -> ()  [unwired: 1 in, 2 out]
      }
      event "Get Fluorophore": Value Change {
        n1961 = event-data() -> ("OldVal"=w2877:bool)  [unwired: 1 in, 4 out]
        n1962 = case shown="True" w2877 {
          selector: w2877 -> [_ w2878]
          frame False {
          }
          frame True {
            n1963 = property on="Move to Position 3" class="Bool"("Val(Sgnl)"=w2878) -> ()  [unwired: 2 in, 2 out]
            n1964 = case shown="1" "Numeric" {
              frame 0, Default {
              }
              frame 1 {
                n1965 = property on="Green Laser ON" class="Bool (strict)"("Val(Sgnl)"=TRUE ("Value (Signaling)")) -> ()  [unwired: 2 in, 2 out]
              }
              frame 2 {
                n1966 = property on="Red Laser ON" class="Bool (strict)"("Val(Sgnl)"=TRUE) -> ()  [unwired: 2 in, 2 out]
              }
            }
          }
        }
      }
      event User Event {
        n1967 = event-data() -> ("Boolean"=w2882:bool)  [unwired: 1 in, 3 out]
        "Green Fluorophore" <- w2882
        n1968 = property on="Get Fluorophore" class="Bool (strict)"("Val(Sgnl)"=w2882) -> ()  [unwired: 2 in, 2 out]
      }
      event User Event {
        n1969 = event-data() -> ("Boolean"=w2883:bool)  [unwired: 1 in, 3 out]
        "Red Fluorophore" <- w2883
        n1970 = property on="Get Fluorophore" class="Bool (strict)"("Val(Sgnl)"=w2883) -> ()  [unwired: 2 in, 2 out]
      }
    }
    n1971 = property on="Get Fluorophore" class="Bool (strict)"("Val(Sgnl)"="Get Fluorophore") -> ()  [unwired: 2 in, 2 out]
    n1972 = Wait (ms)(milliseconds to wait=u32 100) -> ()  [unwired: 1 out]
    n1973 = local read "Stop All"() -> (w2866:bool)
    n1974 = Or(x=w2866, y="stop") -> (x .or. y?=w2867:bool)
  }
  n1975 = timed-loop "Mouse control: trap position (AOM deflection), set confocal spot from image" {
    tunnel: [w2885] -> w208
    tunnel: w18 -> [w2884]
    timing: w130 -> [_]
    timing-out: [_] -> w129
    stop <- w2885 stop-if-true
    n1976 = node-c288() -> ()  [unwired: 2 out]
    n1977 = event shown="[0] \"Pane\": Mouse Down" {
      selector: _ -> [_ _]
      dyn-events: _ -> [_ _]
      timeout: _ -> [_ _]
      tunnel: w2884 -> [w2888 _]
      event Mouse Down {
        n1978 = event-data() -> ("Time"=w2890:u32, "Coords"=w2889:T7, "Button"=w2891:u16)  [unwired: 6 out]
        n1979 = case shown="3" w2891 {
          tunnel: w2890 -> [_ _ w2997]
          tunnel: w2889 -> [_ w2928 w2995]
          tunnel: w2888 -> [_ _ w2993]
          frame 0, Default {
          }
          frame 1 {
            n1980 = property on="APD 2" class="ImageControl"() -> ("Displayed Image Position"=w2898:cluster{"Left":i32, "Top":i32})  [unwired: 2 in, 2 out]
            n1981 = property on="APD 1" class="ImageControl"() -> ("Displayed Image Position"=w2927:cluster{"Left":i32, "Top":i32})  [unwired: 2 in, 2 out]
            n1982 = property on="Detection Laser X" class="ImageControl"() -> ("Displayed Image Position"=w2924:cluster{"Left":i32, "Top":i32})  [unwired: 2 in, 2 out]
            n1983 = property on="Detection Laser Y" class="ImageControl"() -> ("Displayed Image Position"=w2923:cluster{"Left":i32, "Top":i32})  [unwired: 2 in, 2 out]
            n1984 = property on="APD 2" class="ImageControl"() -> ("Displayed Image Size"=w2897:cluster{"Width":u32, "Height":u32})  [unwired: 2 in, 2 out]
            n1985 = property on="APD 1" class="ImageControl"() -> ("Displayed Image Size"=w2925:cluster{"Width":u32, "Height":u32})  [unwired: 2 in, 2 out]
            n1986 = property on="Detection Laser X" class="ImageControl"() -> ("Displayed Image Size"=w2926:cluster{"Width":u32, "Height":u32})  [unwired: 2 in, 2 out]
            n1987 = property on="Detection Laser Y" class="ImageControl"() -> ("Displayed Image Size"=w2922:cluster{"Width":u32, "Height":u32})  [unwired: 2 in, 2 out]
            n1988 = Unbundle By Name(w2897) -> ("Width"=w2894:u32, "Height"=w2893:u32)
            n1989 = Unbundle By Name(w2898) -> ("Left"=w2896:i32, "Top"=w2895:i32)
            n1990 = Unbundle By Name(w2925) -> ("Width"=w2919:u32, "Height"=w2918:u32)
            n1991 = Unbundle By Name(w2926) -> ("Width"=w2915:u32, "Height"=w2914:u32)
            n1992 = Unbundle By Name(w2922) -> ("Width"=w2911:u32, "Height"=w2910:u32)
            n1993 = Unbundle By Name(w2927) -> ("Left"=w2921:i32, "Top"=w2920:i32)
            n1994 = Unbundle By Name(w2924) -> ("Left"=w2917:i32, "Top"=w2916:i32)
            n1995 = Unbundle By Name(w2923) -> ("Left"=w2913:i32, "Top"=w2912:i32)
            n1996 = Bundle("Left"=w2896, "Top"=w2895, "Width"=w2894, "Height"=w2893) -> (w2892:T33)  [unwired: 1 in]
            n1997 = Bundle("Left"=w2921, "Top"=w2920, "Width"=w2919, "Height"=w2918) -> (w2909:T33)  [unwired: 1 in]
            n1998 = Bundle("Left"=w2917, "Top"=w2916, "Width"=w2915, "Height"=w2914) -> (w2908:T33)  [unwired: 1 in]
            n1999 = Bundle("Left"=w2913, "Top"=w2912, "Width"=w2911, "Height"=w2910) -> (w2907:T33)  [unwired: 1 in]
            n2000 = Build Cluster Array(w2892, w2909, w2908, w2907) -> (w2906:T34)
            n2001 = for {
              tunnel: w2928 -> [w2939]
              tunnel: w2906 -> [w2940] mode=indexing
              shift-right: [w2937] -> w2904
              shift-left: TRUE -> [w2938]
              shift-right: [w2936] -> w2902
              shift-left: _ -> [w2932]
              shift-right: [w2935] -> w2901
              shift-left: _ -> [w2931]
              shift-right: [w2934] -> w2900
              shift-left: _ -> [w2930]
              shift-right: [w2933] -> w2899